vi "HFRR ADV v040.vi"() -> ()   [LabVIEW 2025] (continued)
          }
        }
      }
      event "FF BACK", "FF BACK 2", "FF BACK 3", "FF BACK 4", "FF BACK 5", "FF BACK 6": Value Change {
        n806 = event-data() -> ()  [unwired: 1 in, 6 out]
        n807 = stacked-sequence {
          frame #0 {
            n808 = Wait (ms)(milliseconds to wait=u32 1500) -> ()  [unwired: 1 out]
          }
          frame #1 {
            n809 = local write "Due Write"("VC;0") -> ()
          }
          frame #2 {
            n810 = Wait (ms)(milliseconds to wait=u32 1500) -> ()  [unwired: 1 out]
          }
          frame #3 {
            n811 = local write "Due Write"("VC;0") -> ()
          }
          frame #4 {
            w843 = FALSE
            n812 = local write "FF BACK 2"(w843) -> ()
            n813 = local write "FF BACK 3"(w843) -> ()
            n814 = local write "FF BACK 4"(w843) -> ()
            n815 = local write "FF BACK 5"(w843) -> ()
            n816 = local write "FF BACK 6"(w843) -> ()
            n817 = local write "FF BACK"(w843) -> ()
          }
          frame #5 {
            n818 = local write "Temperature Selection"(T13."Default" ("Temperature Selection")) -> ()
            n819 = local write "Calibration Selection"(T8."Default" ("Calibration Selection")) -> ()
            n820 = local write "Friction Force Tab"(T25."Page 1" ("Friction Force Tab")) -> ()
            n821 = local write "Main Calibration Tab"(T7."Main" ("Main Calibration Tab")) -> ()
          }
        }
      }
      event "FF CONTINUE": Value Change {
        n822 = event-data() -> ()  [unwired: 1 in, 6 out]
        n823 = local write "FF CONTINUE"(FALSE ("FF CONTINUE")) -> ()
        n824 = local write "Friction Force Tab"(T25."Page 2" ("Friction Force Tab")) -> ()
      }
      event "FF CONTINUE 2": Value Change {
        n825 = event-data() -> ()  [unwired: 1 in, 6 out]
        n826 = local write "FF CONTINUE 2"(FALSE ("FF CONTINUE")) -> ()
        n827 = local write "Friction Force Tab"(T25."Page 3" ("Friction Force Tab")) -> ()
      }
      event "FF CONTINUE 3": Value Change {
        n828 = event-data() -> ()  [unwired: 1 in, 6 out]
        n829 = local write "FF CONTINUE 3"(FALSE ("FF CONTINUE")) -> ()
        n830 = local write "Friction Force Tab"(T25."Page 4" ("Friction Force Tab")) -> ()
      }
      event "FF CONTINUE 4": Value Change {
        n831 = event-data() -> ()  [unwired: 1 in, 6 out]
        n832 = local write "FF CONTINUE 4"(FALSE ("FF CONTINUE")) -> ()
        n833 = local write "Friction Force Tab"(T25."Page 5" ("Friction Force Tab")) -> ()
      }
      event "FF CONTINUE 5": Value Change {
        n834 = event-data() -> ()  [unwired: 1 in, 6 out]
        n835 = local write "FF CONTINUE 5"(FALSE ("FF CONTINUE")) -> ()
        n836 = local write "Friction Force Tab"(T25."Page 6" ("Friction Force Tab")) -> ()
      }
      event "Stroke Report Button": Value Change {
        n837 = event-data() -> ()  [unwired: 1 in, 6 out]
        n838 = local read "Point 5 - 1.0 mm"() -> (w859:bool)
        n839 = case shown="False" w859 {
          tunnel: [0.8 1.0] -> w858
          frame False {
          }
          frame True {
          }
        }
        n840 = local read "Machine Serial Number"() -> (w862:string)
        n841 = local read "USERNAME"() -> (w860:string)
        n842 = local write "Stroke Report Button"(FALSE ("Stroke Report Button")) -> ()
        n843 = call "Stroke Calibration Report.vi"("measured_value"=w858, "operator_name"=w860, "Instrument_serial Number"=w862) -> ()  [unwired: 7 in, 2 out]
      }
      event "Sample Report Button": Value Change {
        n844 = event-data() -> ()  [unwired: 1 in, 6 out]
        n845 = local read "Machine Serial Number"() -> (w868:string)
        n846 = local read "Sample 0deg temp"() -> (w865:dbl)
        n847 = local read "Sample 60deg temp"() -> (w866:dbl)
        n848 = local read "USERNAME"() -> (w867:string)
        n849 = call "Temperature Calibration Report.vi"("measured_60"=w866, "measured_zero"=w865, "operator_name"=w867, "Instrument_serial Number"=w868) -> ()  [unwired: 6 in, 2 out]
        n850 = local write "Sample Report Button"(FALSE ("Sample Report Button")) -> ()
      }
      event "Air Temperature Report Button": Value Change {
        n851 = event-data() -> ()  [unwired: 1 in, 6 out]
        n852 = local read "Machine Serial Number"() -> (w874:string)
        n853 = local read "Air 0deg temp"() -> (w871:dbl)
        n854 = local read "Air 60deg temp"() -> (w872:dbl)
        n855 = local read "USERNAME"() -> (w873:string)
        n856 = call "Air Temperature Calibration Report.vi"("measured_60"=w872, "measured_zero"=w871, "operator_name"=w873, "Instrument_serial Number"=w874) -> ()  [unwired: 6 in, 2 out]
        n857 = local write "Air Temperature Report Button"(FALSE ("Sample Report Button")) -> ()
      }
      event "Quit": Value Change {
        n858 = event-data() -> ()  [unwired: 1 in, 6 out]
      }
    }
    n859 = Wait (ms)(milliseconds to wait=u32 100) -> ()  [unwired: 1 out]
  }
  n860 = while {
    shift-right: [w877] -> _
    shift-left: "Enum - Selector" -> [w878]
    stop <- w879 stop-if-true
    # "Auto Start Logic Loop"
    n861 = case shown="\"close\"" w878 {
      tunnel: [w882 w888 w915 w947 w977 Auto_Start_enum."Exit" ("Enum - Selector") Auto_Start_enum."Init" ("Enum - Selector")] -> w877
      frame "Init", Default {
        n862 = local read "Auto Start Test"() -> (w881:bool)
        n863 = Select(t=Auto_Start_enum."Humidity & Temperature On" ("Enum - Selector"), s=w881, f=Auto_Start_enum."Init") -> (s? t:f=w882:T15)
      }
      frame "Humidity & Temperature On" {
        n864 = stacked-sequence {
          tunnel: [_ _ _ _ _ _ Auto_Start_enum."Reach point" ("Enum - Selector")] -> w885
          frame #0 {
            w890 = T19."Disabled and Grayed Out" ("Disabled")
            w891 = TRUE ("Heater Button")
            n865 = property on="Humidity" class="Bool (strict)"("DisabledEnum"=w890) -> ()  [unwired: 2 in, 2 out]
            n866 = property on="Heater Button" class="Bool (strict)"("DisabledEnum"=w890) -> ()  [unwired: 2 in, 2 out]
            n867 = local write "Heater Button"(w891) -> ()
            n868 = local write "Humidity"(w891) -> ()
            n869 = property on="Heater Button" class="Bool (strict)"("Val(Sgnl)"=TRUE ("Value (Signaling)")) -> ()  [unwired: 2 in, 2 out]
          }
          frame #1 {
            n870 = Wait (ms)(milliseconds to wait=u32 3000) -> ()  [unwired: 1 out]
          }
          frame #2 {
            n871 = local read "Set Temp"() -> (w897:dbl)
            n872 = Number To Fractional String(number=w897, precision (6)=i16 2) -> (F-format string=w894:string)  [unwired: 2 in]
            n873 = Concatenate Strings("ST;" ("Command"), w894) -> (w895:string)
            n874 = local write "Due Write"(w895) -> ()
          }
          frame #3 {
            n875 = Wait (ms)(milliseconds to wait=u32 1500) -> ()  [unwired: 1 out]
          }
          frame #4 {
            (unwired) i16 2 ("precision (6)")
            n876 = local read "WriteHumidity"() -> (w899:string[])
            n877 = local read "Set Rh"() -> (w902:dbl)
            n878 = Number To Fractional String(number=w902) -> (F-format string=w903:string)  [unwired: 3 in]
            n879 = Concatenate Strings("M;" ("new element/subarray"), w903) -> (w904:string)
            n880 = Insert Into Array(array=w899, new element=w904) -> (w900:string[])  [unwired: 1 in]
            n881 = local write "WriteHumidity"(w900) -> ()
            n882 = local write "Due Write"("HE;1" ("Command")) -> ()
          }
          frame #5 {
            n883 = Wait (ms)(milliseconds to wait=u32 1500) -> ()  [unwired: 1 out]
          }
          frame #6 {
            w907 = TRUE ("Reach point temp")
            n884 = local write "Reach point Humidity"(w907) -> ()
            n885 = local write "Reach point temp"(w907) -> ()
          }
        }
        n886 = local read "Auto Start Test"() -> (w887:bool)
        n887 = Not(x=w887) -> (.not. x?=w886:bool)
        n888 = Select(t=Auto_Start_enum."close", s=w886, f=w885) -> (s? t:f=w888:T15)
      }
      frame "Reach point" {
        w916 = TRUE ("PAUSE")
        w924 = 1.0 ("y")
        w927 = 1.0 ("y")
        n889 = local read "Set Temp"() -> (w909:dbl)
        n890 = local read "Set Humidity:"() -> (w923:dbl)
        n891 = local read "Humidity ( %RH )"() -> (w928:dbl)
        n892 = Add(x=w909, y=w927) -> (x+y=w926:dbl)
        n893 = Subtract(x=w909, y=w927) -> (x-y=w925:dbl)
        n894 = Add(x=w923, y=w924) -> (x+y=w922:dbl)
        n895 = Subtract(x=w923, y=w924) -> (x-y=w921:dbl)
        n896 = local read "TEMP"() -> (w929:dbl)
        n897 = In Range and Coerce(upper limit=w922, x=w928, lower limit=w921) -> (In Range?=w910:bool)  [unwired: 1 out]
        n898 = In Range and Coerce(upper limit=w926, x=w929, lower limit=w925) -> (In Range?=w911:bool)  [unwired: 1 out]
        n899 = case shown="True" w910 {
          frame False {
          }
          frame True {
            n900 = case shown="True" "Reach point Humidity" {
              selector: "Reach point Humidity" -> [_ w935]
              frame False {
              }
              frame True {
                n901 = local read "EVENT LOG"() -> (w932:string)
                n902 = Not(x=w935) -> (.not. x?=w934:bool)
                n903 = local write "Reach point Humidity"(w934) -> ()
                n904 = call "Event Log.vi"("Content"="Target Humidity reached", "EVENT LOG"=w932) -> ("EVENT LOG"=w933:string)  [unwired: 8 in, 1 out]
                n905 = local write "EVENT LOG"(w933) -> ()
              }
            }
          }
        }
        n906 = case shown="True" w911 {
          frame False {
          }
          frame True {
            n907 = case shown="True" "Reach point temp" {
              selector: "Reach point temp" -> [_ w941]
              frame False {
              }
              frame True {
                n908 = local read "EVENT LOG"() -> (w938:string)
                n909 = Not(x=w941) -> (.not. x?=w940:bool)
                n910 = local write "Reach point temp"(w940) -> ()
                n911 = call "Event Log.vi"("Content"="Target Temperature reached", "EVENT LOG"=w938) -> ("EVENT LOG"=w939:string)  [unwired: 8 in, 1 out]
                n912 = local write "EVENT LOG"(w939) -> ()
              }
            }
          }
        }
        n913 = local read "Auto Start Test"() -> (w914:bool)
        n914 = And(x=w911, y=w910) -> (x .and. y?=w920:bool)
        n915 = Select(t=Auto_Start_enum."Maintain Stage" ("Enum - Selector"), s=w920, f=Auto_Start_enum."Reach point" ("Enum - Selector")) -> (s? t:f=w917:T15)
        n916 = Not(x=w914) -> (.not. x?=w913:bool)
        n917 = Select(t=Auto_Start_enum."close", s=w913, f=w917) -> (s? t:f=w915:T15)
        n918 = call "ELAPSED TIMER VI.vi"("RESET"=w916, "PAUSE"=w916) -> ()  [unwired: 7 in, 3 out]
      }
      frame "Maintain Stage" {
        w956 = 2.0 ("y")
        w955 = 1.0 ("y")
        # "Humidity and  temperatures Set Point  have been reached"
        n919 = local read "Set Temp"() -> (w942:dbl)
        n920 = local read "Set Humidity:"() -> (w959:dbl)
        n921 = local read "Humidity ( %RH )"() -> (w962:dbl)
        n922 = Add(x=w942, y=w955) -> (x+y=w961:dbl)
        n923 = Subtract(x=w942, y=w955) -> (x-y=w960:dbl)
        n924 = local read "TEMP"() -> (w963:dbl)
        n925 = Add(x=w959, y=w956) -> (x+y=w958:dbl)
        n926 = Subtract(x=w959, y=w956) -> (x-y=w957:dbl)
        n927 = In Range and Coerce(upper limit=w961, x=w963, lower limit=w960) -> (In Range?=w954:bool)  [unwired: 1 out]
        n928 = In Range and Coerce(upper limit=w958, x=w962, lower limit=w957) -> (In Range?=w953:bool)  [unwired: 1 out]
        n929 = And(x=w954, y=w953) -> (x .and. y?=w952:bool)
        n930 = Not(x=w952) -> (.not. x?=w951:bool)
        n931 = call "ELAPSED TIMER VI.vi"("TARGET"=60.0, "RESET"=w951, "PAUSE"=FALSE) -> ("ELAPSED INDICATION"=w948:bool)  [unwired: 6 in, 2 out]
        n932 = case shown="True" w948 {
          tunnel: w948 -> [_ w966]
          tunnel: [Auto_Start_enum."Maintain Stage" ("Enum - Selector") w965] -> w946
          frame False {
          }
          frame True {
            n933 = stacked-sequence {
              tunnel: w966 -> [_ _ _ _ _]
              tunnel: [_ _ _ _ Auto_Start_enum."Start Stage" ("Enum - Selector")] -> w965
              frame #0 {
                n934 = local read "EVENT LOG"() -> (w968:string)
                n935 = call "Event Log.vi"("Content"="Humidity and temperature set point has stabilized.", "EVENT LOG"=w968) -> ("EVENT LOG"=w969:string)  [unwired: 8 in, 1 out]
                n936 = local write "EVENT LOG"(w969) -> ()
              }
              frame #1 {
                n937 = Wait (ms)(milliseconds to wait=u32 100) -> ()  [unwired: 1 out]
              }
              frame #2 {
                n938 = local read "EVENT LOG"() -> (w972:string)
                n939 = call "Event Log.vi"("Content"="Auto Test Started", "EVENT LOG"=w972) -> ("EVENT LOG"=w973:string)  [unwired: 8 in, 1 out]
                n940 = local write "EVENT LOG"(w973) -> ()
              }
              frame #3 {
                w974 = TRUE ("RUN")
                n941 = local write "RUN"(w974) -> ()
                n942 = property on="Auto Start Temp" class="Bool (strict)"("Val(Sgnl)"=w974) -> ()  [unwired: 2 in, 2 out]
                "Auto Start Temp" <- w974
              }
              frame #4 {
              }
            }
          }
        }
        n943 = local read "Auto Start Test"() -> (w945:bool)
        n944 = Not(x=w945) -> (.not. x?=w944:bool)
        n945 = Select(t=Auto_Start_enum."close", s=w944, f=w946) -> (s? t:f=w947:T15)
      }
      frame "Start Stage" {
        w976 = TRUE ("PAUSE")
        n946 = local read "Auto Start Test"() -> (w981:bool)
        n947 = Not(x=w981) -> (.not. x?=w980:bool)
        n948 = Select(t=Auto_Start_enum."close" ("Enum - Selector"), s=w980, f=Auto_Start_enum."Start Stage" ("Enum - Selector")) -> (s? t:f=w977:T15)
        n949 = call "ELAPSED TIMER VI.vi"("RESET"=w976, "PAUSE"=w976) -> ()  [unwired: 7 in, 3 out]
      }
      frame "close" {
        w984 = FALSE ("Heater Button")
        n950 = local write "RUN"(w984) -> ()
        n951 = local write "Heater Button"(w984) -> ()
        n952 = local write "Humidity"(w984) -> ()
        n953 = local write "Auto Start Test"(w984) -> ()
        n954 = property on="Heater Button" class="Bool (strict)"("Val(Sgnl)"=FALSE ("Value (Signaling)")) -> ()  [unwired: 2 in, 2 out]
        n955 = local write "Humidity 2"(TRUE ("Humidity")) -> ()
      }
      frame "Exit" {
      }
    }
    n956 = Wait (ms)(milliseconds to wait=u32 100) -> ()  [unwired: 1 out]
    n957 = local read "Quit"() -> (w879:bool)
  }
  n958 = property on="Service Password Log" class="Str"("Visible"=w23) -> ()  [unwired: 2 in, 2 out]
  n959 = property on="Password 3" class="Clust (strict)"("Visible"=w23) -> ()  [unwired: 2 in, 2 out]
  n960 = while {
    stop <- w1013 stop-if-true
    w996 = errorcluster {"status"=FALSE, "code"=0, "source"=""} ("error in (no error) 3")
    # "this loop is for manual report generation"
    n961 = local read "Confirm Measrurement"() -> (w995:bool)
    n962 = case shown="True" w995 {
      selector: w995 -> [_ w1103]
      tunnel: errorcluster {"status"=FALSE, "code"=0, "source"=""} ("error in (no error) 3") -> [_ w1104]
      tunnel: [_ w1102] -> _
      frame False {
      }
      frame True {
        n963 = stacked-sequence {
          tunnel: w1104 -> [_ w1137 _]
          tunnel: w1103 -> [_ _ w1244]
          tunnel: [_ w1125 _] -> w1102
          frame #0 {
            n964 = String To Path(string="C:\\LAB-IQ\\Image Calibrate v01.dcf") -> (path=w1107:path)
            n965 = Open/Create/Replace File ("Open File")(file path (use dialog)=w1107) -> (refnum out=w1108:refnum<file>)  [unwired: 5 in, 2 out]
            n966 = for {
              N: 4 -> [_]
              tunnel: w1108 -> [w1114]
              i -> [w1110]
              n967 = Read from Text File ("Read File")(file (use dialog)=w1114) -> (text=w1115:string)  [unwired: 3 in, 3 out]
              n968 = String Subset(string=w1115, offset (0)=6, length (rest)=10 ("length (rest)")) -> (substring=w1111:string)
              n969 = Fract/Exp String To Number(string=w1111) -> (number=w1109:dbl)  [unwired: 3 in, 1 out]
              n970 = case shown="3" w1110 {
                tunnel: w1109 -> [w1116 w1117 _ w1118 _]
                frame 0 {
                  n971 = local write "5x Gain"(w1116) -> ()
                }
                frame 1 {
                  n972 = local write "10x Gain"(w1117) -> ()
                }
                frame 2 {
                }
                frame 3 {
                  n973 = local write "100x gain"(w1118) -> ()
                }
                frame 4, Default {
                }
              }
            }
          }
          frame #1 {
            n974 = local read "TEST STANDARD"() -> (w1120:T3)
            n975 = case shown="\"ISO 12156\"" w1120 {
              tunnel: ["ASTM D6079" "ISO 12156"] -> w1119
              frame "ASTM D6079", Default {
              }
              frame "ISO 12156" {
              }
            }
            n976 = call "IMAGE ANALYSIS.vi"("Enum"=POST_ANALYSIS_ENUM."GET MEASUREMENTS", "error in"=w1137) -> ("error out"=w1144:errorcluster)  [unwired: 8 in, 1 out]
            n977 = local read "Magnification :"() -> (w1130:string)
            n978 = call "Stall Data Flow.vim"("value in"=w1144, "milliseconds to wait"=u32 1000) -> ("value out"=w1143:errorcluster)  [unwired: 1 out]
            n979 = local read "Test File List :"() -> (w1141:string)
            n980 = case shown="\"10x\"" w1130 {
              tunnel: [w1180 w1181] -> w1128
              frame "5x", Default {
                n981 = local read "5x Gain"() -> (w1180:dbl)
              }
              frame "10x" {
                # "5x"
                n982 = local read "10x Gain"() -> (w1181:dbl)
              }
            }
            n983 = call "IMAGE ANALYSIS.vi"("Enum"=POST_ANALYSIS_ENUM."READ", "error in"=w1143) -> ("error out"=w1140:errorcluster, "data out"=w1131:string)  [unwired: 8 in]
            n984 = Match Pattern(string=w1131, regular expression="\"type\": ") -> (after substring=w1135:string)  [unwired: 1 in, 3 out]
            n985 = call "IMAGE PATH CREATION PY.vi"("error in (no error)"=w1140, "File Name :"=w1141) -> ("error out"=w1139:errorcluster, "File Path"=w1127:path, "File Path String:"=w1122:string)  [unwired: 7 in]
            n986 = Match Pattern(string=w1135, regular expression=",") -> (before substring=w1121:string)  [unwired: 1 in, 3 out]
            n987 = local read "Calibration Tab"() -> (w1124:enum32{"Measrument", "Calibrate"})
            n988 = call "Stall Data Flow.vim"("value in"=w1139, "milliseconds to wait"=u32 250) -> ("value out"=w1123:errorcluster)  [unwired: 1 out]
            n989 = Equal?(x=w1121, y="\"rectangle\"") -> (x = y?=w1132:bool)
            n990 = case shown="False" w1132 {
              tunnel: w1131 -> [w1186 w1241]
              tunnel: w1128 -> [_ w1232]
              tunnel: cluster{"major":dbl, "minor":dbl, "average":dbl} {"major"=0.0, "minor"=0.0, "average"=0.0} -> [w1184 w1228]
              tunnel: [w1183 w1225] -> w1126
              tunnel: w1121 -> [w1185 _]
              tunnel: w1128 -> [w1182 _]
              frame False {
                n991 = Equal?(x=w1185, y="\"line\"") -> (x = y?=w1187:bool)
                n992 = case shown="True" w1187 {
                  tunnel: w1186 -> [_ w1202]
                  tunnel: w1184 -> [w1189 w1201]
                  tunnel: [w1189 w1199] -> w1183
                  tunnel: w1182 -> [_ w1198]
                  frame False {
                  }
                  frame True {
                    w1197 = 0.0 ("Major Axis")
                    n993 = Match Pattern(string=w1202, regular expression="\"length_px\":") -> (after substring=w1200:string)  [unwired: 1 in, 3 out]
                    n994 = property on="Major Axis" class="DigNum (strict)"("Caption.Text"="") -> ()  [unwired: 2 in, 2 out]
                    n995 = property on="Minor Axis" class="DigNum (strict)"("Caption.Text"="") -> ()  [unwired: 2 in, 2 out]
                    n996 = property on="Average" class="DigNum (strict)"("Caption.Text"="Line") -> ()  [unwired: 2 in, 2 out]
                    n997 = Fract/Exp String To Number(string=w1200, default (0 dbl)=0.0 ("default (0 DBL)")) -> (number=w1196:dbl)  [unwired: 2 in, 1 out]
                    "Pixel Value" <- w1196
                    n998 = Multiply(x=w1196, y=w1198) -> (x*y=w1209:dbl)
                    n999 = Multiply(x=w1209, y=1000.0) -> (x*y=w1192:dbl)
                    n1000 = Divide(x=w1192, y=1000.0) -> (x/y=w1195:dbl)
                    n1001 = local write "Measurment (mm)"(w1195) -> ()
                    n1002 = Bundle By Name(cluster=w1201, "average"=w1192) -> (w1199:cluster{"major":dbl, "minor":dbl, "average":dbl})
                    n1003 = Number To Fractional String(number=w1192, precision (6)=i16 1) -> (F-format string=w1191:string)  [unwired: 2 in]
                    n1004 = local write "Minor Axis"(w1197) -> ()
                    n1005 = local write "Major Axis"(w1197) -> ()
                    n1006 = Fract/Exp String To Number(string=w1191) -> (number=w1190:dbl)  [unwired: 3 in, 1 out]
                    n1007 = local write "Average"(w1190) -> ()
                  }
                }
              }
              frame True {
                w1229 = 1000.0 ("y")
                w1235 = 0.0 ("default (0 DBL)")
                n1008 = Match Pattern(string=w1241, regular expression=" \"width_px\":") -> (after substring=w1239:string)  [unwired: 1 in, 3 out]
                n1009 = Match Pattern(string=w1239, regular expression="\"height_px\":") -> (before substring=w1237:string, after substring=w1236:string)  [unwired: 1 in, 2 out]
                n1010 = Fract/Exp String To Number(string=w1237, default (0 dbl)=w1235) -> (number=w1234:dbl)  [unwired: 2 in, 1 out]
                n1011 = Fract/Exp String To Number(string=w1236, default (0 dbl)=w1235) -> (number=w1233:dbl)  [unwired: 2 in, 1 out]
                n1012 = Multiply(x=w1234, y=w1232) -> (x*y=w1231:dbl)
                n1013 = Multiply(x=w1233, y=w1232) -> (x*y=w1230:dbl)
                n1014 = Multiply(x=w1231, y=w1229) -> (x*y=w1215:dbl)
                n1015 = Multiply(x=w1230, y=w1229) -> (x*y=w1213:dbl)
                n1016 = Add(x=w1215, y=w1213) -> (x+y=w1227:dbl)
                n1017 = property on="Major Axis" class="DigNum (strict)"("Caption.Text"="Major Axis") -> ()  [unwired: 2 in, 2 out]
                n1018 = property on="Minor Axis" class="DigNum (strict)"("Caption.Text"="Minor Axis") -> ()  [unwired: 2 in, 2 out]
                n1019 = property on="Average" class="DigNum (strict)"("Caption.Text"="Average") -> ()  [unwired: 2 in, 2 out]
                n1020 = Divide(x=w1227, y=2.0) -> (x/y=w1211:dbl)
                n1021 = Bundle By Name(cluster=w1228, "major"=w1215, "minor"=w1213, "average"=w1211) -> (w1225:cluster{"major":dbl, "minor":dbl, "average":dbl})
                n1022 = Number To Fractional String(number=w1213, precision (6)=i16 1) -> (F-format string=w1220:string)  [unwired: 2 in]
                n1023 = Number To Fractional String(number=w1211, precision (6)=i16 1) -> (F-format string=w1221:string)  [unwired: 2 in]
                n1024 = Number To Fractional String(number=w1215, precision (6)=i16 1) -> (F-format string=w1219:string)  [unwired: 2 in]
                n1025 = Fract/Exp String To Number(string=w1220) -> (number=w1212:dbl)  [unwired: 3 in, 1 out]
                n1026 = Fract/Exp String To Number(string=w1221) -> (number=w1210:dbl)  [unwired: 3 in, 1 out]
                n1027 = Fract/Exp String To Number(string=w1219) -> (number=w1214:dbl)  [unwired: 3 in, 1 out]
                n1028 = local write "Major Axis"(w1214) -> ()
                n1029 = local write "Average"(w1210) -> ()
                n1030 = local write "Minor Axis"(w1212) -> ()
              }
            }
            n1031 = case shown="\"Measrument\", Default" w1124 {
              tunnel: w1127 -> [w1154 _]
              tunnel: w1126 -> [w1153 _]
              tunnel: [w1150 w1179] -> w1125
              tunnel: w1123 -> [w1152 w1179]
              tunnel: w1122 -> [w1151 _]
              tunnel: w1119 -> [w1149 _]
              frame "Measrument", Default {
                n1032 = stacked-sequence {
                  tunnel: w1154 -> [w1172 _]
                  tunnel: w1153 -> [w1170 _]
                  tunnel: w1152 -> [w1168 _]
                  tunnel: w1151 -> [w1167 _]
                  tunnel: [w1162 _] -> w1150
                  tunnel: w1149 -> [w1155 _]
                  frame #0 {
                    n1033 = call "IMAGE ANALYSIS.vi"("Enum"=POST_ANALYSIS_ENUM."SAVE IMAGE", "error in"=w1168, "IMAGE FILE PATH"=w1167) -> ("error out"=w1166:errorcluster)  [unwired: 7 in, 1 out]
                    n1034 = call "Stall Data Flow.vim"("value in"=w1166, "milliseconds to wait"=u32 1000) -> ("value out"=w1157:errorcluster)  [unwired: 1 out]
                    n1035 = local read "Test File List :"() -> (w1174:string)
                    n1036 = call "IMAGE ANALYSIS.vi"("Enum"=POST_ANALYSIS_ENUM."MINIMIZE UI", "error in"=w1157) -> ("error out"=w1164:errorcluster)  [unwired: 8 in, 1 out]
                    n1037 = Bundle By Name(cluster=T27 {"File Name"="", "Test Method"="", "Operator"="", "Fuel Description"="", "Date and time"=""} ("Main Ref"), "Test Method"=w1155, "File Name"=w1174) -> (w1175:T27)
                    n1038 = call "Stall Data Flow.vim"("value in"=w1164, "milliseconds to wait"=u32 1500) -> ("value out"=w1159:errorcluster)  [unwired: 1 out]
                    n1039 = call "duf file read.vi"("error in (no error)"=w1159, "Main Ref"=w1175) -> ("error out"=w1173:errorcluster, "Main Ref 2"=w1171:T27)  [unwired: 8 in]
                    n1040 = call "DETECTION REPORT for manual.vi"("error in (no error)"=w1173, "return value 3"=w1170, "Image File Path"=w1172, "Main Ref"=w1171) -> ("error out"=w1169:errorcluster)  [unwired: 7 in]
                    n1041 = call <vilib>:"Clear Errors.vi"("error in (no error)"=w1169) -> ("error out"=w1160:errorcluster)  [unwired: 5 in, 1 out]
                    n1042 = call "IMAGE ANALYSIS.vi"("Enum"=POST_ANALYSIS_ENUM."MINIMIZE UI", "error in"=w1160) -> ("error out"=w1162:errorcluster)  [unwired: 8 in, 1 out]
                  }
                  frame #1 {
                    n1043 = local write "Main Tab"(T2."HOME" ("Main Tab")) -> ()
                    n1044 = local write "Main Dashboard Buttons"(T1."Home" ("Main Dashboard Buttons")) -> ()
                  }
                }
              }
              frame "Calibrate" {
              }
            }
          }
          frame #2 {
            n1045 = Not(x=w1244) -> (.not. x?=w1243:bool)
            n1046 = local write "Confirm Measrurement"(w1243) -> ()
            n1047 = local read "Calibration Tab"() -> (w1242:enum32{"Measrument", "Calibrate"})
            n1048 = case shown="\"Measrument\", Default" w1242 {
              frame "Measrument", Default {
                (unwired) T21."HOME" ("Main Tab")
                n1049 = local write "Main Tab"(T2."HOME" ("Main Tab")) -> ()
              }
              frame "Calibrate" {
              }
            }
          }
        }
      }
    }
    n1050 = local read "Humidity"() -> (w987:bool)
    n1051 = local read "Save Change"() -> (w992:bool)
    n1052 = local read "Calibrate"() -> (w993:bool)
    n1053 = local read "Auto Start Test"() -> (w988:bool)
    n1054 = case shown="True" w993 {
      selector: w993 -> [_ w1100]
      frame False {
      }
      frame True {
        n1055 = Not(x=w1100) -> (.not. x?=w1099:bool)
        n1056 = local write "Calibrate"(w1099) -> ()
        n1057 = local write "Calibration Tab"(enum32{"Measrument", "Calibrate"}."Calibrate" ("Calibration Tab")) -> ()
      }
    }
    n1058 = case shown="True" w992 {
      selector: w992 -> [_ w1044]
      frame False {
      }
      frame True {
        n1059 = stacked-sequence {
          tunnel: w1044 -> [_ _ _ _ w1098]
          frame #0 {
            n1060 = call "IMAGE ANALYSIS.vi"("Enum"=POST_ANALYSIS_ENUM."HIDE UI") -> ()  [unwired: 9 in, 2 out]
          }
          frame #1 {
            n1061 = local read "100x gain"() -> (w1046:dbl)
            n1062 = local read "10x Gain"() -> (w1047:dbl)
            n1063 = local read "5x Gain"() -> (w1048:dbl)
            n1064 = Number To Fractional String(number=w1047, width (-)=i16 4, precision (6)=i16 7) -> (F-format string=w1069:string)  [unwired: 1 in]
            n1065 = Number To Fractional String(number=0.0, width (-)=i16 4, precision (6)=i16 7) -> (F-format string=w1064:string)  [unwired: 1 in]
            n1066 = Number To Fractional String(number=w1046, width (-)=i16 4, precision (6)=i16 7) -> (F-format string=w1052:string)  [unwired: 1 in]
            n1067 = Number To Fractional String(number=w1048, width (-)=i16 10 ("precision (6)"), precision (6)=i16 7) -> (F-format string=w1078:string)  [unwired: 1 in]
            n1068 = Concatenate Strings("[CH1]" ("string"), w1078, " - 5x Gain" ("string"), "\r") -> (w1068:string)
            n1069 = Concatenate Strings("[CH2]" ("string"), w1069, " - 10x Gain" ("string"), "\r") -> (w1067:string)
            n1070 = Concatenate Strings("[CH3]" ("string"), w1064, " - 20x Gain" ("string"), "\r") -> (w1058:string)
            n1071 = Concatenate Strings("[CH4]" ("string"), w1052, " - 100x Gain" ("string"), "\r") -> (w1051:string)
            n1072 = String To Path(string="C:\\LAB-IQ\\Image Calibrate v01.dcf") -> (path=w1081:path)
            n1073 = Concatenate Strings(w1068, w1067, w1058, w1051) -> (w1066:string)
            n1074 = call <vilib>:"Write Characters To File.vi"("append to file? (new file:F)"=FALSE, "character string"=w1066, "file path (dialog if empty)"=w1081) -> ()  [unwired: 2 in, 1 out]
          }
          frame #2 {
            n1075 = String To Path(string="C:\\LAB-IQ\\Image Calibrate v01.dcf") -> (path=w1084:path)
            n1076 = Open/Create/Replace File ("Open File")(file path (use dialog)=w1084) -> (refnum out=w1085:refnum<file>)  [unwired: 5 in, 2 out]
            n1077 = for {
              N: 4 -> [_]
              tunnel: w1085 -> [w1091]
              i -> [w1087]
              n1078 = Read from Text File ("Read File")(file (use dialog)=w1091) -> (text=w1092:string)  [unwired: 3 in, 3 out]
              n1079 = String Subset(string=w1092, offset (0)=6, length (rest)=10 ("length (rest)")) -> (substring=w1088:string)
              n1080 = Fract/Exp String To Number(string=w1088) -> (number=w1086:dbl)  [unwired: 3 in, 1 out]
              n1081 = case shown="3" w1087 {
                tunnel: w1086 -> [w1093 w1094 _ w1095 _]
                frame 0 {
                  n1082 = local write "5x Gain"(w1093) -> ()
                }
                frame 1 {
                  n1083 = local write "10x Gain"(w1094) -> ()
                }
                frame 2 {
                }
                frame 3 {
                  n1084 = local write "100x gain"(w1095) -> ()
                }
                frame 4, Default {
                }
              }
            }
          }
          frame #3 {
            n1085 = call "IMAGE ANALYSIS.vi"("Enum"=POST_ANALYSIS_ENUM."SHOW UI") -> ()  [unwired: 9 in, 2 out]
          }
          frame #4 {
            n1086 = Not(x=w1098) -> (.not. x?=w1097:bool)
            n1087 = local write "Save Change"(w1097) -> ()
          }
        }
      }
    }
    n1088 = case shown="False" w988 {
      tunnel: w987 -> [w1014 _]
      frame False {
        n1089 = case shown="True" w1014 {
          frame False {
          }
          frame True {
            n1090 = local read "Set Humidity:"() -> (w1018:dbl)
            n1091 = local read "Set Humidity:"() -> (w1021:dbl)
            n1092 = local read "Humidity ( %RH )"() -> (w1022:dbl)
            n1093 = Subtract(x=w1018, y=2.0) -> (x-y=w1016:dbl)
            n1094 = Add(x=w1021, y=2.0) -> (x+y=w1017:dbl)
            n1095 = In Range and Coerce(upper limit=w1017, x=w1022, lower limit=w1016) -> (In Range?=w1015:bool)  [unwired: 1 out]
            n1096 = case shown="True" w1015 {
              frame False {
              }
              frame True {
                n1097 = case shown="True" "Manual Humididty Reached" {
                  selector: "Manual Humididty Reached" -> [_ w1025]
                  frame False {
                  }
                  frame True {
                    n1098 = Not(x=w1025) -> (.not. x?=w1024:bool)
                    n1099 = local write "Manual Humididty Reached"(w1024) -> ()
                    n1100 = local read "EVENT LOG"() -> (w1027:string)
                    n1101 = call "Event Log.vi"("Content"="Target Humidity reached", "EVENT LOG"=w1027) -> ("EVENT LOG"=w1026:string)  [unwired: 8 in, 1 out]
                    n1102 = local write "EVENT LOG"(w1026) -> ()
                  }
                }
              }
            }
          }
        }
      }
      frame True {
        n1103 = local write "Manual Humididty Reached"(TRUE ("Manual Humididty Reached")) -> ()
      }
    }
    n1104 = local read "Cap Live Image"() -> (w1008:bool)
    n1105 = local read "SCAR MEASURMENT"() -> (w1011:enum32{"Auto Scar", "Manual Scar"})
    n1106 = Equal?(x=w1011, y=enum32{"Auto Scar", "Manual Scar"}."Manual Scar" ("SCAR MEASURMENT")) -> (x = y?=w1009:bool)
    n1107 = And(x=w1009, y=w1008) -> (x .and. y?=w1007:bool)
    n1108 = Wait (ms)(milliseconds to wait=u32 250) -> ()  [unwired: 1 out]
    n1109 = case shown="True" w1007 {
      selector: w1007 -> [_ w1330]
      frame False {
      }
      frame True {
        n1110 = stacked-sequence {
          tunnel: [_ _ _ w1349 _] -> _
          tunnel: w1330 -> [_ _ _ _ w1356]
          frame #0 {
            w1331 = 0.0
            n1111 = local write "Major Axis"(w1331) -> ()
            n1112 = local write "Minor Axis"(w1331) -> ()
            n1113 = local write "Average"(w1331) -> ()
          }
          frame #1 {
            n1114 = call "CAMERA LIVE FEED FGV.vi"("Enum - Menu"=CAMERA_LIVE_FEED_ENUM."CAMERA MINIMIZE") -> ()  [unwired: 9 in, 2 out]
          }
          frame #2 {
            n1115 = local read "Magnification len live scar"() -> (w1335:string)
            n1116 = case shown="\"10x\", Default" w1335 {
              tunnel: ["_10x" "_5x"] -> w1334
              frame "10x", Default {
              }
              frame "5x" {
              }
            }
            n1117 = local read "FILE 3"() -> (w1341:string)
            n1118 = call <vilib>:"Trim Whitespace.vi"("string"="C:\\LAB-IQ\\images\\") -> ("trimmed string"=w1343:string)  [unwired: 1 in]
            n1119 = String To Path(string=w1343) -> (path=w1342:path)
            n1120 = Concatenate Strings(w1341, w1334, ".png" ("string")) -> (w1340:string)
            n1121 = Build Path(base path=w1342, name or relative path=w1340) -> (appended path=w1339:path)
            n1122 = Path To String(path=w1339) -> (string=w1338:string)
            n1123 = call "CAMERA LIVE FEED FGV.vi"("Enum - Menu"=CAMERA_LIVE_FEED_ENUM."CAMERA SAVE", "Image Path"=w1338) -> ("error out"=w1336:errorcluster)  [unwired: 8 in, 1 out]
            n1124 = case shown="No Error" w1336 {
              frame No Error {
                n1125 = One Button Dialog(message="Image saved successfully") -> ()  [unwired: 1 in, 1 out]
              }
              frame Error {
              }
            }
          }
          frame #3 {
            n1126 = call "LIST FILE NAMES.vi"() -> ("error out"=w1351:errorcluster, "filenames"=w1348:string[])  [unwired: 10 in]
            n1127 = call "IMAGE ANALYSIS.vi"("Enum"=POST_ANALYSIS_ENUM."SHOW UI", "error in"=w1351) -> ("error out"=w1349:errorcluster)  [unwired: 8 in, 1 out]
            n1128 = property on="Test File List :" class="CmbBox"("Strings[]"=w1348) -> ()  [unwired: 2 in, 2 out]
          }
          frame #4 {
            (unwired) T26."Report" ("Main Dashboard Buttons")
            (unwired) T28."Report" ("Main Dashboard Buttons")
            n1129 = Not(x=w1356) -> (.not. x?=w1355:bool)
            n1130 = local write "Zoom Factore"(0.0 ("Zoom Factore")) -> ()
            n1131 = local write "Cap Live Image"(w1355) -> ()
            n1132 = local write "Main Tab"(T2."Adv Scar Report" ("Main Tab")) -> ()
            n1133 = property on="Cap Live Image" class="Bool (strict)"("BoolText.Text"="Capture Image" ("Boolean Text.Text")) -> ()  [unwired: 2 in, 2 out]
            n1134 = local write "Main Dashboard Buttons"(T1."Report" ("Main Dashboard Buttons")) -> ()
          }
        }
      }
    }
    n1135 = local read "change Gain"() -> (w991:bool)
    n1136 = local read "Back Square"() -> (w990:bool)
    n1137 = case shown="True" w991 {
      selector: w991 -> [_ w1035]
      frame False {
      }
      frame True {
        n1138 = stacked-sequence {
          tunnel: w1035 -> [_ w1043]
          frame #0 {
            n1139 = local read "Actual (µm)"() -> (w1039:dbl)
            n1140 = local read "Pixel Value"() -> (w1038:dbl)
            n1141 = local read "Magnification :"() -> (w1037:string)
            n1142 = Divide(x=w1039, y=w1038) -> (x/y=w1036:dbl)
            n1143 = case shown="\"10x\"" w1037 {
              tunnel: w1036 -> [w1040 w1041]
              frame "10x" {
                n1144 = local write "10x Gain"(w1040) -> ()
              }
              frame "5x", Default {
                n1145 = local write "5x Gain"(w1041) -> ()
              }
            }
          }
          frame #1 {
            n1146 = Not(x=w1043) -> (.not. x?=w1042:bool)
            n1147 = local write "change Gain"(w1042) -> ()
          }
        }
      }
    }
    n1148 = case shown="True" w990 {
      selector: w990 -> [_ w1033]
      frame False {
      }
      frame True {
        n1149 = Not(x=w1033) -> (.not. x?=w1032:bool)
        n1150 = local write "Back Square"(w1032) -> ()
        n1151 = local write "Calibration Tab"(enum32{"Measrument", "Calibrate"}."Measrument" ("Calibration Tab")) -> ()
      }
    }
    n1152 = local read "Rectangle Tool"() -> (w1002:bool)
    n1153 = local read "Clear ROI Tool"() -> (w1001:bool)
    n1154 = local read "Open Image"() -> (w1006:bool)
    n1155 = local read "line tool"() -> (w1003:bool)
    n1156 = local read "OUT"() -> (w1004:bool)
    n1157 = local read "In"() -> (w1005:bool)
    n1158 = case shown="True" w1006 {
      selector: w1006 -> [_ w1316]
      tunnel: [w1307 w1318] -> _
      tunnel: w996 -> [w1307 w1317]
      frame False {
      }
      frame True {
        w1311 = "_5x" ("regular expression")
        n1159 = Not(x=w1316) -> (.not. x?=w1315:bool)
        n1160 = local write "Open Image"(w1315) -> ()
        n1161 = call "IMAGE ANALYSIS.vi"("Enum"=POST_ANALYSIS_ENUM."HIDE UI", "error in"=w1317) -> ("error out"=w1325:errorcluster)  [unwired: 8 in, 1 out]
        n1162 = call <vilib>:"Clear Errors.vi"("error in (no error)"=w1325) -> ("error out"=w1308:errorcluster)  [unwired: 5 in, 1 out]
        n1163 = call "File Dialog"("start path"=path "C:/LAB-IQ/images", "error in"=w1308) -> ("selected path"=w1310:path, "error out"=w1323:errorcluster)  [unwired: 10 in, 2 out]
        "Image path  2" <- w1310
        n1164 = call <vilib>:"Clear Errors.vi"("error in (no error)"=w1323) -> ("error out"=w1322:errorcluster)  [unwired: 5 in, 1 out]
        n1165 = call "IMAGE ANALYSIS.vi"("Enum"=POST_ANALYSIS_ENUM."OPEN FILE", "error in"=w1322, "File Path"=w1310) -> ("error out"=w1321:errorcluster)  [unwired: 7 in, 1 out]
        n1166 = call <vilib>:"Clear Errors.vi"("error in (no error)"=w1321) -> ("error out"=w1320:errorcluster)  [unwired: 5 in, 1 out]
        n1167 = call "IMAGE ANALYSIS.vi"("Enum"=POST_ANALYSIS_ENUM."SHOW UI", "error in"=w1320) -> ("error out"=w1318:errorcluster)  [unwired: 8 in, 1 out]
        n1168 = local write "Zoom Factore"(100.0 ("Zoom Factore")) -> ()
        n1169 = Strip Path(path=w1310) -> (name=w1313:string)  [unwired: 1 out]
        n1170 = Match Pattern(string=w1313, regular expression=w1311) -> (match substring=w1312:string)  [unwired: 1 in, 3 out]
        n1171 = Equal?(x=w1312, y=w1311) -> (x = y?=w1309:bool)
        n1172 = case shown="False" w1309 {
          frame False {
            n1173 = local write "Magnification :"("10x" ("Magnification :")) -> ()
          }
          frame True {
            n1174 = local write "Magnification :"("5x" ("Magnification :")) -> ()
          }
        }
      }
    }
    n1175 = case shown="True" w1004 {
      selector: w1004 -> [_ w1292]
      tunnel: w996 -> [w1289 w1297]
      tunnel: [w1289 w1291] -> _
      frame False {
      }
      frame True {
        n1176 = Not(x=w1292) -> (.not. x?=w1290:bool)
        n1177 = local read "Zoom Factore"() -> (w1295:dbl)
        n1178 = local write "OUT"(w1290) -> ()
        n1179 = call "IMAGE ANALYSIS.vi"("Enum"=POST_ANALYSIS_ENUM."ZOOM OUT", "error in"=w1297) -> ("error out"=w1291:errorcluster)  [unwired: 8 in, 1 out]
        n1180 = Divide(x=w1295, y=1.2) -> (x/y=w1293:dbl)
        n1181 = local write "Zoom Factore"(w1293) -> ()
      }
    }
    n1182 = case shown="True" w1005 {
      selector: w1005 -> [_ w1301]
      tunnel: w996 -> [w1298 w1306]
      tunnel: [w1298 w1299] -> _
      frame False {
      }
      frame True {
        n1183 = Not(x=w1301) -> (.not. x?=w1300:bool)
        n1184 = local read "Zoom Factore"() -> (w1304:dbl)
        n1185 = local write "In"(w1300) -> ()
        n1186 = call "IMAGE ANALYSIS.vi"("Enum"=POST_ANALYSIS_ENUM."ZOOM IN", "error in"=w1306) -> ("error out"=w1299:errorcluster)  [unwired: 8 in, 1 out]
        n1187 = Multiply(x=w1304, y=1.2) -> (x*y=w1302:dbl)
        n1188 = local write "Zoom Factore"(w1302) -> ()
      }
    }
    n1189 = case shown="True" w1001 {
      selector: w1001 -> [_ w1273]
      tunnel: w996 -> [w1271 w1275]
      tunnel: [w1271 w1274] -> _
      frame False {
      }
      frame True {
        n1190 = Not(x=w1273) -> (.not. x?=w1272:bool)
        n1191 = local write "Clear ROI Tool"(w1272) -> ()
        n1192 = call "IMAGE ANALYSIS.vi"("Enum"=POST_ANALYSIS_ENUM."CLEAR ROI", "error in"=w1275) -> ("error out"=w1274:errorcluster)  [unwired: 8 in, 1 out]
      }
    }
    n1193 = case shown="True" w1003 {
      selector: w1003 -> [_ w1285]
      tunnel: w996 -> [w1283 w1288]
      tunnel: [w1283 w1286] -> _
      frame False {
      }
      frame True {
        n1194 = Not(x=w1285) -> (.not. x?=w1284:bool)
        n1195 = local write "line tool"(w1284) -> ()
        n1196 = call "IMAGE ANALYSIS.vi"("Enum"=POST_ANALYSIS_ENUM."DRAW LINE", "error in"=w1288) -> ("error out"=w1286:errorcluster)  [unwired: 8 in, 1 out]
      }
    }
    n1197 = case shown="True" w1002 {
      selector: w1002 -> [_ w1279]
      tunnel: w996 -> [w1277 w1281]
      tunnel: [w1277 w1280] -> _
      frame False {
      }
      frame True {
        n1198 = Not(x=w1279) -> (.not. x?=w1278:bool)
        n1199 = local write "Rectangle Tool"(w1278) -> ()
        n1200 = call "IMAGE ANALYSIS.vi"("Enum"=POST_ANALYSIS_ENUM."DRAW REC", "error in"=w1281) -> ("error out"=w1280:errorcluster)  [unwired: 8 in, 1 out]
      }
    }
    n1201 = local read "SCAR MEASURMENT"() -> (w989:enum32{"Auto Scar", "Manual Scar"})
    n1202 = local read "Fit to Screen Tool"() -> (w998:bool)
    n1203 = local read "Resize Tool"() -> (w997:bool)
    n1204 = case shown="\"Manual Scar\", Default" w989 {
      frame "Auto Scar" {
        n1205 = property on="Cap Live Image" class="Bool (strict)"("BoolText.Text"="Report" ("Boolean Text.Text")) -> ()  [unwired: 2 in, 2 out]
      }
      frame "Manual Scar", Default {
        n1206 = property on="Cap Live Image" class="Bool (strict)"("BoolText.Text"="Save Image" ("Boolean Text.Text")) -> ()  [unwired: 2 in, 2 out]
      }
    }
    n1207 = local read "ROI Color Tool"() -> (w999:bool)
    n1208 = local read "Pan Tool"() -> (w1000:bool)
    n1209 = case shown="True" w1000 {
      selector: w1000 -> [_ w1267]
      tunnel: w996 -> [w1265 w1269]
      tunnel: [w1265 w1268] -> _
      frame False {
      }
      frame True {
        n1210 = Not(x=w1267) -> (.not. x?=w1266:bool)
        n1211 = call "IMAGE ANALYSIS.vi"("Enum"=POST_ANALYSIS_ENUM."PAN", "error in"=w1269) -> ("error out"=w1268:errorcluster)  [unwired: 8 in, 1 out]
        n1212 = local write "Pan Tool"(w1266) -> ()
      }
    }
    n1213 = case shown="True" w997 {
      selector: w997 -> [_ w1251]
      tunnel: w996 -> [w1246 w1248]
      tunnel: [w1246 w1247] -> _
      frame False {
      }
      frame True {
        n1214 = Not(x=w1251) -> (.not. x?=w1250:bool)
        n1215 = local write "Resize Tool"(w1250) -> ()
        n1216 = call "IMAGE ANALYSIS.vi"("Enum"=POST_ANALYSIS_ENUM."RESIZE MODE", "error in"=w1248) -> ("error out"=w1247:errorcluster)  [unwired: 8 in, 1 out]
      }
    }
    n1217 = case shown="True" w998 {
      selector: w998 -> [_ w1256]
      tunnel: [w1252 w1257] -> _
      tunnel: w996 -> [w1252 w1255]
      frame False {
      }
      frame True {
        n1218 = Not(x=w1256) -> (.not. x?=w1254:bool)
        n1219 = local write "Zoom Factore"(100.0 ("Zoom Factore")) -> ()
        n1220 = local write "Fit to Screen Tool"(w1254) -> ()
        n1221 = call "IMAGE ANALYSIS.vi"("Enum"=POST_ANALYSIS_ENUM."FIT", "error in"=w1255) -> ("error out"=w1257:errorcluster)  [unwired: 8 in, 1 out]
      }
    }
    n1222 = case shown="True" w999 {
      selector: w999 -> [_ w1262]
      tunnel: [w1259 w1263] -> _
      tunnel: w996 -> [w1259 w1260]
      frame False {
      }
      frame True {
        n1223 = Not(x=w1262) -> (.not. x?=w1261:bool)
        n1224 = local write "ROI Color Tool"(w1261) -> ()
        n1225 = call "IMAGE ANALYSIS.vi"("Enum"=POST_ANALYSIS_ENUM."SET ROI COLOR", "error in"=w1260) -> ("error out"=w1263:errorcluster)  [unwired: 8 in, 1 out]
      }
    }
    n1226 = local read "Quit"() -> (w1013:bool)
  }
  n1227 = while {
    stop <- w1358 stop-if-true
    n1228 = local read "Image Path"() -> (w1361:path)
    n1229 = local read "Print 3"() -> (w1364:bool)
    n1230 = Equal?(x=w1361, y=path "") -> (x = y?=w1360:bool)
    n1231 = Not(x=w1360) -> (.not. x?=w1359:bool)
    n1232 = property on="Print 3" class="Bool (strict)"("Visible"=w1359) -> ()  [unwired: 2 in, 2 out]
    n1233 = case shown="True" w1364 {
      frame False {
        n1234 = local write "Rd"(TRUE ("Boolean 7")) -> ()
      }
      frame True {
        n1235 = flat-sequence {
          tunnel: [w1404] -> w1372
          tunnel: [w1391] -> w1370
          tunnel: [w1401] -> w1366
          tunnel: w1372 -> [w1413]
          tunnel: [w1413] -> w1371
          tunnel: w1370 -> [w1412]
          tunnel: [w1412] -> w1369
          tunnel: [w1410] -> w1368
          tunnel: [w1409] -> w1367
          tunnel: w1366 -> [w1409]
          tunnel: w1371 -> [w1415]
          tunnel: w1369 -> [w1416]
          tunnel: w1368 -> [_]
          tunnel: w1367 -> [w1414]
          frame #0 {
            n1236 = case shown="True" "Rd" {
              frame False {
              }
              frame True {
                n1237 = while {
                  tunnel: "abcdefABCDEF" ("string 2") -> [w1383]
                  shift-right: [w1381] -> w1375
                  shift-left: "" -> [w1380]
                  i -> [w1390]
                  stop <- w1389 stop-if-true
                  n1238 = Random Number (0-1)() -> (number: 0 to 1=w1384:dbl)
                  n1239 = Multiply(x=w1384, y=62.0) -> (x*y=w1386:dbl)
                  n1240 = Decrement(x="Length 2") -> (x-1=w1379:i16)
                  n1241 = To Word Integer(number=w1386) -> (16bit integer=w1387:i16)
                  n1242 = String Subset(string=w1383, offset (0)=w1387, length (rest)=1 ("length (rest)")) -> (substring=w1382:string)
                  n1243 = Greater Or Equal?(x=w1390, y=w1379) -> (x >= y?=w1389:bool)
                  n1244 = Concatenate Strings(w1382, w1380) -> (w1381:string)
                }
                "String 10" <- w1375
                n1245 = local write "Rd"(FALSE ("Boolean 7")) -> ()
              }
            }
          }
          frame #1 {
            w1402 = "_resized.jpg" ("command line")
            (unwired) ".jpg -resize 320x240 " ("string")
            (unwired) "Choose an Image File" ("prompt")
            # "-resize 1798x425"
            n1246 = local read "Image Path"() -> (w1396:path)
            n1247 = Strip Path(path=w1396) -> (stripped path=w1391:path, name=w1392:string)
            n1248 = Match Pattern(string=w1392, regular expression=".jpg") -> (before substring=→"before substring 2":string, after substring=→"after substring":string)  [unwired: 1 in, 2 out]
            n1249 = Match Pattern(string=w1392, regular expression="\\") -> (before substring=w1398:string)  [unwired: 1 in, 3 out]
            n1250 = Match Pattern(string=w1398, regular expression=".jpg") -> (before substring=w1397:string)  [unwired: 1 in, 3 out]
            n1251 = Concatenate Strings("cmd /c convert " ("string"), w1397, ".jpg -resize 320x240  " ("command line"), w1397, w1402) -> (w1405:string)
            n1252 = call <vilib>:"System Exec.vi"("run minimized? (F)"=TRUE, "wait until completion? (T)"=TRUE, "working directory"=w1391, "command line"=w1405) -> ("error out"=w1404:errorcluster)  [unwired: 4 in, 3 out]
            "error out 2" <- w1404
            n1253 = Concatenate Strings(w1397, w1402) -> (w1401:string)
          }
          frame #2 {
            n1254 = Wait (ms)(milliseconds to wait=u32 2000 ("millisecond timer value")) -> (millisecond timer value=w1410:u32)
          }
          frame #3 {
            n1255 = case shown="No Error" w1415 {
              tunnel: w1416 -> [w1419 _]
              tunnel: w1414 -> [w1417 _]
              frame No Error {
                (unwired) ".jpg" ("string")
                n1256 = Path To String(path=w1419) -> (string=w1423:string)
                n1257 = Concatenate Strings(w1423, "\\" ("string"), w1417) -> (w1422:string)
                n1258 = String To Path(string=w1422) -> (path=w1421:path)
                n1259 = call <vilib>:"Read JPEG File.vi"("path to JPEG file"=w1421) -> ("image data"=w1425:T16)  [unwired: 8 in, 2 out]
                "image data" <- w1425
                n1260 = local write "Print 3"(FALSE ("Print 2")) -> ()
                n1261 = call <vilib>:"Draw Flattened Pixmap.vi"("image data"=w1425) -> ("new picture"=→"new picture":picture)  [unwired: 8 in]
              }
              frame Error {
              }
            }
          }
        }
      }
    }
    n1262 = Wait (ms)(milliseconds to wait=u32 20 ("millisecond timer value")) -> ()  [unwired: 1 out]
    n1263 = local read "Quit"() -> (w1358:bool)
  }
  n1264 = while {
    tunnel: w40 -> [_]
    tunnel: w26 -> [_]
    stop <- w1455 stop-if-true
    # "New Adv Logics"
    n1265 = local read "Main Tab"() -> (w1436:T2)
    n1266 = local read "Main Tab"() -> (w1453:T2)
    n1267 = local read "Sign In"() -> (w1452:bool)
    n1268 = case shown="\"Adv Scar\"" w1436 {
      frame "HOME", Default {
        n1269 = local read "LIVE FEED MIN TEMP"() -> (w1588:bool)
        n1270 = local write "LIVE FEED MAX TEMP"(TRUE ("LIVE FEED MAX TEMP")) -> ()
        n1271 = local read "CAMERA ROI MIN TEMP"() -> (w1586:bool)
        n1272 = case shown="True" w1588 {
          selector: w1588 -> [_ w1595]
          frame False {
          }
          frame True {
            n1273 = Not(x=w1595) -> (.not. x?=w1594:bool)
            n1274 = local write "LIVE FEED MIN TEMP"(w1594) -> ()
            n1275 = call "CAMERA LIVE FEED FGV.vi"("Enum - Menu"=CAMERA_LIVE_FEED_ENUM."CAMERA MINIMIZE") -> ()  [unwired: 9 in, 2 out]
          }
        }
        n1276 = case shown="True" w1586 {
          selector: w1586 -> [_ w1592]
          frame False {
          }
          frame True {
            n1277 = Not(x=w1592) -> (.not. x?=w1591:bool)
            n1278 = local write "CAMERA ROI MIN TEMP"(w1591) -> ()
            n1279 = call "IMAGE ANALYSIS.vi"("Enum"=POST_ANALYSIS_ENUM."MINIMIZE UI") -> ()  [unwired: 9 in, 2 out]
          }
        }
        n1280 = local write "CAMERA ROI MAX TEMP"(TRUE ("CAMERA ROI MAX TEMP")) -> ()
      }
      frame "Test Setup" {
        n1281 = local read "LIVE FEED MIN TEMP"() -> (w1598:bool)
        n1282 = local read "CAMERA ROI MIN TEMP"() -> (w1596:bool)
        n1283 = local write "LIVE FEED MAX TEMP"(TRUE ("LIVE FEED MAX TEMP")) -> ()
        n1284 = case shown="True" w1598 {
          selector: w1598 -> [_ w1605]
          frame False {
          }
          frame True {
            n1285 = Not(x=w1605) -> (.not. x?=w1604:bool)
            n1286 = local write "LIVE FEED MIN TEMP"(w1604) -> ()
            n1287 = call "CAMERA LIVE FEED FGV.vi"("Enum - Menu"=CAMERA_LIVE_FEED_ENUM."CAMERA MINIMIZE") -> ()  [unwired: 9 in, 2 out]
          }
        }
        n1288 = case shown="True" w1596 {
          selector: w1596 -> [_ w1602]
          frame False {
          }
          frame True {
            n1289 = Not(x=w1602) -> (.not. x?=w1601:bool)
            n1290 = local write "CAMERA ROI MIN TEMP"(w1601) -> ()
            n1291 = call "IMAGE ANALYSIS.vi"("Enum"=POST_ANALYSIS_ENUM."MINIMIZE UI") -> ()  [unwired: 9 in, 2 out]
          }
        }
        n1292 = local write "CAMERA ROI MAX TEMP"(TRUE ("CAMERA ROI MAX TEMP")) -> ()
      }
      frame "Acquire" {
        n1293 = local read "LIVE FEED MIN TEMP"() -> (w1608:bool)
        n1294 = local write "LIVE FEED MAX TEMP"(TRUE ("LIVE FEED MAX TEMP")) -> ()
        n1295 = local read "CAMERA ROI MIN TEMP"() -> (w1606:bool)
        n1296 = case shown="True" w1608 {
          selector: w1608 -> [_ w1615]
          frame False {
          }
          frame True {
            n1297 = Not(x=w1615) -> (.not. x?=w1614:bool)
            n1298 = local write "LIVE FEED MIN TEMP"(w1614) -> ()
            n1299 = call "CAMERA LIVE FEED FGV.vi"("Enum - Menu"=CAMERA_LIVE_FEED_ENUM."CAMERA MINIMIZE") -> ()  [unwired: 9 in, 2 out]
          }
        }
        n1300 = case shown="True" w1606 {
          selector: w1606 -> [_ w1612]
          frame False {
          }
          frame True {
            n1301 = Not(x=w1612) -> (.not. x?=w1611:bool)
            n1302 = local write "CAMERA ROI MIN TEMP"(w1611) -> ()
            n1303 = call "IMAGE ANALYSIS.vi"("Enum"=POST_ANALYSIS_ENUM."MINIMIZE UI") -> ()  [unwired: 9 in, 2 out]
          }
        }
        n1304 = local write "CAMERA ROI MAX TEMP"(TRUE ("CAMERA ROI MAX TEMP")) -> ()
      }
      frame "Adv Scar" {
        n1305 = local read "CAMERA ROI MIN TEMP"() -> (w1616:bool)
        n1306 = case shown="True" "LIVE FEED MAX TEMP" {
          selector: "LIVE FEED MAX TEMP" -> [_ w1637]
          frame False {
          }
          frame True {
            n1307 = Not(x=w1637) -> (.not. x?=w1636:bool)
            n1308 = local write "LIVE FEED MAX TEMP"(w1636) -> ()
            n1309 = call "CAMERA LIVE FEED FGV.vi"("Enum - Menu"=CAMERA_LIVE_FEED_ENUM."CAMERA RESTORE") -> ("error out"=w1627:errorcluster)  [unwired: 9 in, 1 out]
            n1310 = Type Cast(type=30, x=0) -> (*(type *) &x=w1631:i32)
            n1311 = Add(x=w1631, y=48) -> (x+y=w1632:i32)
            n1312 = call "CAMERA LIVE FEED FGV.vi"("Enum - Menu"=CAMERA_LIVE_FEED_ENUM."CAMERA MODE SET", "error in (no error)"=w1627, "CAMERA MODE"=w1632) -> ("error out"=w1624:errorcluster)  [unwired: 7 in, 1 out]
            n1313 = call "CAMERA LIVE FEED FGV.vi"("Enum - Menu"=CAMERA_LIVE_FEED_ENUM."CAMERA GRAY", "error in (no error)"=w1624) -> ("error out"=w1623:errorcluster)  [unwired: 8 in, 1 out]
            n1314 = call "LIST FILE NAMES.vi"("error in (no error)"=w1623) -> ("error out"=w1633:errorcluster, "filenames"=w1634:string[])  [unwired: 9 in]
            n1315 = property on="FILE 3" class="CmbBox"(error in=w1633, "Strings[]"=w1634) -> ()  [unwired: 1 in, 2 out]
          }
        }
        n1316 = case shown="True" w1616 {
          selector: w1616 -> [_ w1622]
          frame False {
          }
          frame True {
            n1317 = Not(x=w1622) -> (.not. x?=w1621:bool)
            n1318 = local write "CAMERA ROI MIN TEMP"(w1621) -> ()
            n1319 = call "IMAGE ANALYSIS.vi"("Enum"=POST_ANALYSIS_ENUM."MINIMIZE UI") -> ()  [unwired: 9 in, 2 out]
          }
        }
        n1320 = local write "CAMERA ROI MAX TEMP"(TRUE ("CAMERA ROI MAX TEMP")) -> ()
        "LIVE FEED MIN TEMP" <- TRUE ("LIVE FEED MIN TEMP")
      }
      frame "Adv Scar Report" {
        n1321 = local read "CAMERA ROI MAX TEMP"() -> (w1638:bool)
        n1322 = local read "LIVE FEED MIN TEMP"() -> (w1640:bool)
        n1323 = local write "LIVE FEED MAX TEMP"(TRUE ("LIVE FEED MAX TEMP")) -> ()
        n1324 = case shown="True" w1640 {
          selector: w1640 -> [_ w1649]
          frame False {
          }
          frame True {
            n1325 = Not(x=w1649) -> (.not. x?=w1648:bool)
            n1326 = local write "LIVE FEED MIN TEMP"(w1648) -> ()
            n1327 = call "CAMERA LIVE FEED FGV.vi"("Enum - Menu"=CAMERA_LIVE_FEED_ENUM."CAMERA MINIMIZE") -> ()  [unwired: 9 in, 2 out]